vi "SaccadeAnalyser - Main.vi"(8 "error in (no error)":errorcluster, 11 "Data IN":T3={"Impulse Positions"=[{"Start"=5471, "End"=5813, "Impulse Plane"=enum."Yaw", "Impulse Direction +ve?"=FALSE, "Time offset"=0, "Amplitude offset"=0.0}, {"Start"=6974, "End"=7325, "Impulse Plane"=enum."Yaw", "Impulse Direction +ve?"=TRUE, "Time offset"=0, "Amplitude offset"=0.0}, {"Start"=7641, "End"=7980, "Impulse Plane"=enum."Yaw", "Impulse Direction +ve?"=FALSE, "Time offset"=0, "Amplitude offset"=0.0}, {"Start"=9060, "End"=9400, "Impulse Plane"=enum."Yaw", "Impulse Direction +ve?"=FALSE, "Time offset"=0, "Amplitude offset"=0.0}, {"Start"=9938, "End"=10282, "Impulse Plane"=enum."Yaw", "Impulse Direction +ve?"=FALSE, "Time offset"=0, "Amplitude offset"=0.0}, {"Start"=10800, "End"=11142, "Impulse Plane"=enum."Yaw", "Impulse Direction +ve?"=FALSE, "Time offset"=0, "Amplitude offset"=0.0}, {"Start"=11602, "End"=11942, "Impulse Plane"=enum."Yaw", "Impulse Direction +ve?"=TRUE, "Time offset"=0, "Amplitude offset"=0.0}, {"Start"=12449, "End"=12790, "Impulse Plane"=enum."Yaw", "Impulse Direction +ve?"=TRUE, "Time offset"=0, "Amplitude offset"=0.0}, {"Start"=13310, "End"=13653, "Impulse Plane"=enum."Yaw", "Impulse Direction +ve?"=TRUE, "Time offset"=0, "Amplitude offset"=0.0}, {"Start"=14191, "End"=14535, "Impulse Plane"=enum."Yaw", "Impulse Direction +ve?"=TRUE, "Time offset"=0, "Amplitude offset"=0.0}, {"Start"=15040, "End"=15380, "Impulse Plane"=enum."Yaw", "Impulse Direction +ve?"=FALSE, "Time offset"=0, "Amplitude offset"=0.0}, {"Start"=16780, "End"=17124, "Impulse Plane"=enum."Yaw", "Impulse Direction +ve?"=TRUE, "Time offset"=0, "Amplitude offset"=0.0}, {"Start"=17572, "End"=17913, "Impulse Plane"=enum."Yaw", "Impulse Direction +ve?"=FALSE, "Time offset"=0, "Amplitude offset"=0.0}, {"Start"=18369, "End"=18713, "Impulse Plane"=enum."Yaw", "Impulse Direction +ve?"=FALSE, "Time offset"=0, "Amplitude offset"=0.0}, {"Start"=19174, "End"=19519, "Impulse Plane"=enum."Yaw", "Impulse Direction +ve?"=FALSE, "Time offset"=0, "Amplitude offset"=0.0}, {"Start"=19928, "End"=20270, "Impulse Plane"=enum."Yaw", "Impulse Direction +ve?"=TRUE, "Time offset"=0, "Amplitude offset"=0.0}, {"Start"=20762, "End"=21121, "Impulse Plane"=enum."Yaw", "Impulse Direction +ve?"=FALSE, "Time offset"=0, "Amplitude offset"=0.0}, {"Start"=21554, "End"=21888, "Impulse Plane"=enum."Yaw", "Impulse Direction +ve?"=FALSE, "Time offset"=0, "Amplitude offset"=0.0}, {"Start"=22293, "End"=22639, "Impulse Plane"=enum."Yaw", "Impulse Direction +ve?"=TRUE, "Time offset"=0, "Amplitude offset"=0.0}, {"Start"=23109, "End"=23464, "Impulse Plane"=enum."Yaw", "Impulse Direction +ve?"=TRUE, "Time offset"=0, "Amplitude offset"=0.0}, {"Start"=23868, "End"=24215, "Impulse Plane"=enum."Yaw", "Impulse Direction +ve?"=TRUE, "Time offset"=0, "Amplitude offset"=0.0}, {"Start"=24643, "End"=24992, "Impulse Plane"=enum."Yaw", "Impulse Direction +ve?"=FALSE, "Time offset"=0, "Amplitude offset"=0.0}, {"Start"=25685, "End"=26023, "Impulse Plane"=enum."Yaw", "Impulse Direction +ve?"=FALSE, "Time offset"=0, "Amplitude offset"=0.0}, {"Start"=26431, "End"=26768, "Impulse Plane"=enum."Yaw", "Impulse Direction +ve?"=FALSE, "Time offset"=0, "Amplitude offset"=0.0}, {"Start"=27251, "End"=27595, "Impulse Plane"=enum."Yaw", "Impulse Direction +ve?"=FALSE, "Time offset"=0, "Amplitude offset"=0.0}, {"Start"=28832, "End"=29180, "Impulse Plane"=enum."Yaw", "Impulse Direction +ve?"=TRUE, "Time offset"=0, "Amplitude offset"=0.0}, {"Start"=31028, "End"=31383, "Impulse Plane"=enum."LARP", "Impulse Direction +ve?"=FALSE, "Time offset"=0, "Amplitude offset"=0.0}, {"Start"=32603, "End"=32936, "Impulse Plane"=enum."LARP", "Impulse Direction +ve?"=TRUE, "Time offset"=0, "Amplitude offset"=0.0}, {"Start"=33445, "End"=33779, "Impulse Plane"=enum."LARP", "Impulse Direction +ve?"=TRUE, "Time offset"=0, "Amplitude offset"=0.0}, {"Start"=34276, "End"=34629, "Impulse Plane"=enum."LARP", "Impulse Direction +ve?"=FALSE, "Time offset"=0, "Amplitude offset"=0.0}, {"Start"=35114, "End"=35460, "Impulse Plane"=enum."LARP", "Impulse Direction +ve?"=FALSE, "Time offset"=0, "Amplitude offset"=0.0}, {"Start"=35981, "End"=36324, "Impulse Plane"=enum."LARP", "Impulse Direction +ve?"=TRUE, "Time offset"=0, "Amplitude offset"=0.0}, {"Start"=36920, "End"=37249, "Impulse Plane"=enum."LARP", "Impulse Direction +ve?"=TRUE, "Time offset"=0, "Amplitude offset"=0.0}, {"Start"=37988, "End"=38322, "Impulse Plane"=enum."LARP", "Impulse Direction +ve?"=TRUE, "Time offset"=0, "Amplitude offset"=0.0}, {"Start"=38964, "End"=39324, "Impulse Plane"=enum."LARP", "Impulse Direction +ve?"=FALSE, "Time offset"=0, "Amplitude offset"=0.0}, {"Start"=39948, "End"=40284, "Impulse Plane"=enum."LARP", "Impulse Direction +ve?"=TRUE, "Time offset"=0, "Amplitude offset"=0.0}, {"Start"=40958, "End"=41293, "Impulse Plane"=enum."LARP", "Impulse Direction +ve?"=TRUE, "Time offset"=0, "Amplitude offset"=0.0}, {"Start"=41899, "End"=42229, "Impulse Plane"=enum."LARP", "Impulse Direction +ve?"=TRUE, "Time offset"=0, "Amplitude offset"=0.0}, {"Start"=42801, "End"=43154, "Impulse Plane"=enum."LARP", "Impulse Direction +ve?"=FALSE, "Time offset"=0, "Amplitude offset"=0.0}, {"Start"=43641, "End"=43980, "Impulse Plane"=enum."LARP", "Impulse Direction +ve?"=TRUE, "Time offset"=0, "Amplitude offset"=0.0}, {"Start"=44466, "End"=44821, "Impulse Plane"=enum."LARP", "Impulse Direction +ve?"=FALSE, "Time offset"=0, "Amplitude offset"=0.0}, {"Start"=45388, "End"=45722, "Impulse Plane"=enum."LARP", "Impulse Direction +ve?"=TRUE, "Time offset"=0, "Amplitude offset"=0.0}, {"Start"=46149, "End"=46510, "Impulse Plane"=enum."LARP", "Impulse Direction +ve?"=FALSE, "Time offset"=0, "Amplitude offset"=0.0}, {"Start"=47874, "End"=48206, "Impulse Plane"=enum."LARP", "Impulse Direction +ve?"=TRUE, "Time offset"=0, "Amplitude offset"=0.0}, {"Start"=50143, "End"=50479, "Impulse Plane"=enum."RALP", "Impulse Direction +ve?"=TRUE, "Time offset"=0, "Amplitude offset"=0.0}, {"Start"=50976, "End"=51310, "Impulse Plane"=enum."RALP", "Impulse Direction +ve?"=FALSE, "Time offset"=0, "Amplitude offset"=0.0}, {"Start"=51892, "End"=52226, "Impulse Plane"=enum."RALP", "Impulse Direction +ve?"=FALSE, "Time offset"=0, "Amplitude offset"=0.0}, {"Start"=52839, "End"=53171, "Impulse Plane"=enum."RALP", "Impulse Direction +ve?"=FALSE, "Time offset"=0, "Amplitude offset"=0.0}, {"Start"=53676, "End"=54012, "Impulse Plane"=enum."RALP", "Impulse Direction +ve?"=TRUE, "Time offset"=0, "Amplitude offset"=0.0}, {"Start"=54530, "End"=54877, "Impulse Plane"=enum."RALP", "Impulse Direction +ve?"=FALSE, "Time offset"=0, "Amplitude offset"=0.0}, {"Start"=55371, "End"=55711, "Impulse Plane"=enum."RALP", "Impulse Direction +ve?"=TRUE, "Time offset"=0, "Amplitude offset"=0.0}, {"Start"=56153, "End"=56482, "Impulse Plane"=enum."RALP", "Impulse Direction +ve?"=FALSE, "Time offset"=0, "Amplitude offset"=0.0}, {"Start"=57053, "End"=57390, "Impulse Plane"=enum."RALP", "Impulse Direction +ve?"=FALSE, "Time offset"=0, "Amplitude offset"=0.0}, {"Start"=57954, "End"=58292, "Impulse Plane"=enum."RALP", "Impulse Direction +ve?"=FALSE, "Time offset"=0, "Amplitude offset"=0.0}, {"Start"=58794, "End"=59130, "Impulse Plane"=enum."RALP", "Impulse Direction +ve?"=TRUE, "Time offset"=0, "Amplitude offset"=0.0}, {"Start"=59587, "End"=59931, "Impulse Plane"=enum."RALP", "Impulse Direction +ve?"=TRUE, "Time offset"=0, "Amplitude offset"=0.0}, {"Start"=60399, "End"=60744, "Impulse Plane"=enum."RALP", "Impulse Direction +ve?"=FALSE, "Time offset"=0, "Amplitude offset"=0.0}, {"Start"=61218, "End"=61559, "Impulse Plane"=enum."RALP", "Impulse Direction +ve?"=FALSE, "Time offset"=0, "Amplitude offset"=0.0}, {"Start"=62100, "End"=62442, "Impulse Plane"=enum."RALP", "Impulse Direction +ve?"=FALSE, "Time offset"=0, "Amplitude offset"=0.0}, {"Start"=62989, "End"=63322, "Impulse Plane"=enum."RALP", "Impulse Direction +ve?"=FALSE, "Time offset"=0, "Amplitude offset"=0.0}, {"Start"=63787, "End"=64136, "Impulse Plane"=enum."RALP", "Impulse Direction +ve?"=TRUE, "Time offset"=0, "Amplitude offset"=0.0}, {"Start"=64603, "End"=64953, "Impulse Plane"=enum."RALP", "Impulse Direction +ve?"=FALSE, "Time offset"=0, "Amplitude offset"=0.0}, {"Start"=65462, "End"=65795, "Impulse Plane"=enum."RALP", "Impulse Direction +ve?"=FALSE, "Time offset"=0, "Amplitude offset"=0.0}, {"Start"=66308, "End"=66645, "Impulse Plane"=enum."RALP", "Impulse Direction +ve?"=FALSE, "Time offset"=0, "Amplitude offset"=0.0}, {"Start"=67052, "End"=67402, "Impulse Plane"=enum."RALP", "Impulse Direction +ve?"=TRUE, "Time offset"=0, "Amplitude offset"=0.0}], "No. Imp"=15, "Parameter Time Series"=[{"time offset"=0.0, "Offset"=0.0, "Gain"=1.0, "inverse"=FALSE, "filter data"=FALSE, "dots"=FALSE, "interpolate"=FALSE, "List 1"=5, "Color Box"=6618880, "Boolean"=TRUE}, {"time offset"=0.0, "Offset"=0.0, "Gain"=1.0, "inverse"=FALSE, "filter data"=FALSE, "dots"=FALSE, "interpolate"=FALSE, "List 1"=6, "Color Box"=6618880, "Boolean"=FALSE}, {"time offset"=0.0, "Offset"=0.0, "Gain"=1.0, "inverse"=FALSE, "filter data"=FALSE, "dots"=FALSE, "interpolate"=FALSE, "List 1"=7, "Color Box"=6618880, "Boolean"=FALSE}, {"time offset"=0.0, "Offset"=0.0, "Gain"=1.0, "inverse"=FALSE, "filter data"=FALSE, "dots"=FALSE, "interpolate"=FALSE, "List 1"=13, "Color Box"=16777224, "Boolean"=TRUE}, {"time offset"=0.0, "Offset"=0.0, "Gain"=1.0, "inverse"=FALSE, "filter data"=FALSE, "dots"=FALSE, "interpolate"=FALSE, "List 1"=14, "Color Box"=16777224, "Boolean"=FALSE}, {"time offset"=0.0, "Offset"=0.0, "Gain"=1.0, "inverse"=FALSE, "filter data"=FALSE, "dots"=FALSE, "interpolate"=FALSE, "List 1"=15, "Color Box"=16777224, "Boolean"=FALSE}], "Parameter Impuls Series"=[{"Color"=6618880, "Visible"=TRUE, "Channel"=1, "Invert"=FALSE, "Desaccade"=FALSE, "Offset"=0.0, "Gain"=1.0}, {"Color"=6618880, "Visible"=FALSE, "Channel"=6, "Invert"=FALSE, "Desaccade"=FALSE, "Offset"=0.0, "Gain"=1.0}, {"Color"=6618880, "Visible"=FALSE, "Channel"=7, "Invert"=FALSE, "Desaccade"=FALSE, "Offset"=0.0, "Gain"=1.0}, {"Color"=16777224, "Visible"=TRUE, "Channel"=13, "Invert"=FALSE, "Desaccade"=FALSE, "Offset"=0.0, "Gain"=1.0}, {"Color"=16777224, "Visible"=FALSE, "Channel"=14, "Invert"=FALSE, "Desaccade"=FALSE, "Offset"=0.0, "Gain"=1.0}, {"Color"=16777224, "Visible"=FALSE, "Channel"=15, "Invert"=FALSE, "Desaccade"=FALSE, "Offset"=0.0, "Gain"=1.0}], "Experiment Parameters"={"Freq"=0.0, "Vel"=0, "Acc"=0, "Stimulus"="Head Impulse"}, "Autosort File"=refnum, "Data File"={"Data Channels"=array34x71049[2415666 elements], "Sample Rate"=500, "Channel List"=["Hz Position-in-Head", "Hz Velocity-in-Head", "Hy Position-in-Head", "Hy Velocity-in-Head", "Hx Position-in-Head", "Hx Velocity-in-Head", "Hl Velocity-in-Head", "Hr Velocity-in-Head", "Lx Position-in-Head", "Ly Position-in-Head", "Lz Position-in-Head", "Lx Velocity-in-Head", "Ly Velocity-in-Head", "Lz Velocity-in-Head", "Ll Velocity-in-Head", "Lr Velocity-in-Head", "Rx Position-in-Head", "Ry Position-in-Head", "Rz Position-in-Head", "Rx Velocity-in-Head", "Ry Velocity-in-Head", "Rz Velocity-in-Head", "Rl Velocity-in-Head", "Rr Velocity-in-Head", "Target on/off", "aux input 1", "aux input 2", " ", "", "", "", "Target Hor", "Target Ver", ""]}, "Experiment data path"=path "C:/Users/w.figtree/Desktop/Coils Data/3", "Image data path"=path "/Macintosh HD/Users/patrick/Studium/Diploma Thesis/Data Analysis", "LVS data path"=path "/Macintosh HD/Users/patrick/Studium/Diploma Thesis/Data Analysis", "Raw copy path"=path "/Macintosh HD/Users/patrick/Studium/Diploma Thesis/Data Analysis", "filename"="passive_lvs.lvs", "desaccading parameters"={"Tolerance"=3, "Acc Range"=7000.0, "Sample Rate"=500, "Impulse Plane 2"=enum."Yaw", "Impulse dir"=FALSE}, "Experiment Parameters 2"={"Subject"="SE Trial Short Term", "Strain"="", "Rotation plane"="", "Experimenter"=" ", "Trial"=0.0, "Time"=0.0}, "Excel"={"Excel._Application"=refnum, "Use Excel"=TRUE, "Worksheet SINE"=refnum, "Row SINE"=0, "Worksheet TRANS"=refnum, "Row TRANS"=0}, "Session Config File"=refnum, "Autosort Parameter Set"=4, "EMA Version"="EMA 2016a", "desacc "={"Threshold 1 [Acc]"=7000.0, "Threshold 2 [% of TH1]"=60, "tolerance"=3, "Search WD "=0.1, " always use TH2"=FALSE, "Range"=3.0, "Max time"=120.0, "Min time"=20.0, "Velocity Threshold"=150}, "Cycle Nr for Saccades"={"POS"=0, "NEG"=0}, "calibration name"="u_calibration_1_p00001s001_calib.mat", "Excel"=refnum} {"Parameter Time Series"."time offset" format="%.3f"; "Parameter Time Series"."Gain" format="%.1f"; "Parameter Time Series"."Offset" format="%.1f"; "Parameter Time Series"."List 1" items=["Motor-Pos", "Motor-Vel", "Lx Position-in-Head", "Ly Position-in-Head", "Lz Position-in-Head", "Lx Velocity-in-Head", "Ly Velocity-in-Head", "Lz Velocity-in-Head", "Ll Velocity-in-Head", "Lr Velocity-in-Head", "Lx Accel-in-Head", "Ly Accel-in-Head", "Lz Accel-in-Head", "Rx Position-in-Head", "Ry Position-in-Head", "Rz Position-in-Head", "Rx Velocity-in-Head", "Ry Velocity-in-Head", "Rz Velocity-in-Head", "Rl Velocity-in-Head", "Rr Velocity-in-Head", "Rx Accel-in-Head", "Ry Accel-in-Head", "Rz Accel-in-Head", "Global Trigger", "", "", ""]; "Parameter Impuls Series"."Gain" format="%.1f"; "Parameter Impuls Series"."Offset" format="%.1f"}) -> (0 "error out":errorcluster, 3 "Data OUT":T3={"Impulse Positions"=[{"Start"=5471, "End"=5813, "Impulse Plane"=enum."Yaw", "Impulse Direction +ve?"=FALSE, "Time offset"=0, "Amplitude offset"=0.0}, {"Start"=6974, "End"=7325, "Impulse Plane"=enum."Yaw", "Impulse Direction +ve?"=TRUE, "Time offset"=0, "Amplitude offset"=0.0}, {"Start"=7641, "End"=7980, "Impulse Plane"=enum."Yaw", "Impulse Direction +ve?"=FALSE, "Time offset"=0, "Amplitude offset"=0.0}, {"Start"=9060, "End"=9400, "Impulse Plane"=enum."Yaw", "Impulse Direction +ve?"=FALSE, "Time offset"=0, "Amplitude offset"=0.0}, {"Start"=9938, "End"=10282, "Impulse Plane"=enum."Yaw", "Impulse Direction +ve?"=FALSE, "Time offset"=0, "Amplitude offset"=0.0}, {"Start"=10800, "End"=11142, "Impulse Plane"=enum."Yaw", "Impulse Direction +ve?"=FALSE, "Time offset"=0, "Amplitude offset"=0.0}, {"Start"=11602, "End"=11942, "Impulse Plane"=enum."Yaw", "Impulse Direction +ve?"=TRUE, "Time offset"=0, "Amplitude offset"=0.0}, {"Start"=12449, "End"=12790, "Impulse Plane"=enum."Yaw", "Impulse Direction +ve?"=TRUE, "Time offset"=0, "Amplitude offset"=0.0}, {"Start"=13310, "End"=13653, "Impulse Plane"=enum."Yaw", "Impulse Direction +ve?"=TRUE, "Time offset"=0, "Amplitude offset"=0.0}, {"Start"=14191, "End"=14535, "Impulse Plane"=enum."Yaw", "Impulse Direction +ve?"=TRUE, "Time offset"=0, "Amplitude offset"=0.0}, {"Start"=15040, "End"=15380, "Impulse Plane"=enum."Yaw", "Impulse Direction +ve?"=FALSE, "Time offset"=0, "Amplitude offset"=0.0}, {"Start"=16780, "End"=17124, "Impulse Plane"=enum."Yaw", "Impulse Direction +ve?"=TRUE, "Time offset"=0, "Amplitude offset"=0.0}, {"Start"=17572, "End"=17913, "Impulse Plane"=enum."Yaw", "Impulse Direction +ve?"=FALSE, "Time offset"=0, "Amplitude offset"=0.0}, {"Start"=18369, "End"=18713, "Impulse Plane"=enum."Yaw", "Impulse Direction +ve?"=FALSE, "Time offset"=0, "Amplitude offset"=0.0}, {"Start"=19174, "End"=19519, "Impulse Plane"=enum."Yaw", "Impulse Direction +ve?"=FALSE, "Time offset"=0, "Amplitude offset"=0.0}, {"Start"=19928, "End"=20270, "Impulse Plane"=enum."Yaw", "Impulse Direction +ve?"=TRUE, "Time offset"=0, "Amplitude offset"=0.0}, {"Start"=20762, "End"=21121, "Impulse Plane"=enum."Yaw", "Impulse Direction +ve?"=FALSE, "Time offset"=0, "Amplitude offset"=0.0}, {"Start"=21554, "End"=21888, "Impulse Plane"=enum."Yaw", "Impulse Direction +ve?"=FALSE, "Time offset"=0, "Amplitude offset"=0.0}, {"Start"=22293, "End"=22639, "Impulse Plane"=enum."Yaw", "Impulse Direction +ve?"=TRUE, "Time offset"=0, "Amplitude offset"=0.0}, {"Start"=23109, "End"=23464, "Impulse Plane"=enum."Yaw", "Impulse Direction +ve?"=TRUE, "Time offset"=0, "Amplitude offset"=0.0}, {"Start"=23868, "End"=24215, "Impulse Plane"=enum."Yaw", "Impulse Direction +ve?"=TRUE, "Time offset"=0, "Amplitude offset"=0.0}, {"Start"=24643, "End"=24992, "Impulse Plane"=enum."Yaw", "Impulse Direction +ve?"=FALSE, "Time offset"=0, "Amplitude offset"=0.0}, {"Start"=25685, "End"=26023, "Impulse Plane"=enum."Yaw", "Impulse Direction +ve?"=FALSE, "Time offset"=0, "Amplitude offset"=0.0}, {"Start"=26431, "End"=26768, "Impulse Plane"=enum."Yaw", "Impulse Direction +ve?"=FALSE, "Time offset"=0, "Amplitude offset"=0.0}, {"Start"=27251, "End"=27595, "Impulse Plane"=enum."Yaw", "Impulse Direction +ve?"=FALSE, "Time offset"=0, "Amplitude offset"=0.0}, {"Start"=28832, "End"=29180, "Impulse Plane"=enum."Yaw", "Impulse Direction +ve?"=TRUE, "Time offset"=0, "Amplitude offset"=0.0}, {"Start"=31028, "End"=31383, "Impulse Plane"=enum."LARP", "Impulse Direction +ve?"=FALSE, "Time offset"=0, "Amplitude offset"=0.0}, {"Start"=32603, "End"=32936, "Impulse Plane"=enum."LARP", "Impulse Direction +ve?"=TRUE, "Time offset"=0, "Amplitude offset"=0.0}, {"Start"=33445, "End"=33779, "Impulse Plane"=enum."LARP", "Impulse Direction +ve?"=TRUE, "Time offset"=0, "Amplitude offset"=0.0}, {"Start"=34276, "End"=34629, "Impulse Plane"=enum."LARP", "Impulse Direction +ve?"=FALSE, "Time offset"=0, "Amplitude offset"=0.0}, {"Start"=35114, "End"=35460, "Impulse Plane"=enum."LARP", "Impulse Direction +ve?"=FALSE, "Time offset"=0, "Amplitude offset"=0.0}, {"Start"=35981, "End"=36324, "Impulse Plane"=enum."LARP", "Impulse Direction +ve?"=TRUE, "Time offset"=0, "Amplitude offset"=0.0}, {"Start"=36920, "End"=37249, "Impulse Plane"=enum."LARP", "Impulse Direction +ve?"=TRUE, "Time offset"=0, "Amplitude offset"=0.0}, {"Start"=37988, "End"=38322, "Impulse Plane"=enum."LARP", "Impulse Direction +ve?"=TRUE, "Time offset"=0, "Amplitude offset"=0.0}, {"Start"=38964, "End"=39324, "Impulse Plane"=enum."LARP", "Impulse Direction +ve?"=FALSE, "Time offset"=0, "Amplitude offset"=0.0}, {"Start"=39948, "End"=40284, "Impulse Plane"=enum."LARP", "Impulse Direction +ve?"=TRUE, "Time offset"=0, "Amplitude offset"=0.0}, {"Start"=40958, "End"=41293, "Impulse Plane"=enum."LARP", "Impulse Direction +ve?"=TRUE, "Time offset"=0, "Amplitude offset"=0.0}, {"Start"=41899, "End"=42229, "Impulse Plane"=enum."LARP", "Impulse Direction +ve?"=TRUE, "Time offset"=0, "Amplitude offset"=0.0}, {"Start"=42801, "End"=43154, "Impulse Plane"=enum."LARP", "Impulse Direction +ve?"=FALSE, "Time offset"=0, "Amplitude offset"=0.0}, {"Start"=43641, "End"=43980, "Impulse Plane"=enum."LARP", "Impulse Direction +ve?"=TRUE, "Time offset"=0, "Amplitude offset"=0.0}, {"Start"=44466, "End"=44821, "Impulse Plane"=enum."LARP", "Impulse Direction +ve?"=FALSE, "Time offset"=0, "Amplitude offset"=0.0}, {"Start"=45388, "End"=45722, "Impulse Plane"=enum."LARP", "Impulse Direction +ve?"=TRUE, "Time offset"=0, "Amplitude offset"=0.0}, {"Start"=46149, "End"=46510, "Impulse Plane"=enum."LARP", "Impulse Direction +ve?"=FALSE, "Time offset"=0, "Amplitude offset"=0.0}, {"Start"=47874, "End"=48206, "Impulse Plane"=enum."LARP", "Impulse Direction +ve?"=TRUE, "Time offset"=0, "Amplitude offset"=0.0}, {"Start"=50143, "End"=50479, "Impulse Plane"=enum."RALP", "Impulse Direction +ve?"=TRUE, "Time offset"=0, "Amplitude offset"=0.0}, {"Start"=50976, "End"=51310, "Impulse Plane"=enum."RALP", "Impulse Direction +ve?"=FALSE, "Time offset"=0, "Amplitude offset"=0.0}, {"Start"=51892, "End"=52226, "Impulse Plane"=enum."RALP", "Impulse Direction +ve?"=FALSE, "Time offset"=0, "Amplitude offset"=0.0}, {"Start"=52839, "End"=53171, "Impulse Plane"=enum."RALP", "Impulse Direction +ve?"=FALSE, "Time offset"=0, "Amplitude offset"=0.0}, {"Start"=53676, "End"=54012, "Impulse Plane"=enum."RALP", "Impulse Direction +ve?"=TRUE, "Time offset"=0, "Amplitude offset"=0.0}, {"Start"=54530, "End"=54877, "Impulse Plane"=enum."RALP", "Impulse Direction +ve?"=FALSE, "Time offset"=0, "Amplitude offset"=0.0}, {"Start"=55371, "End"=55711, "Impulse Plane"=enum."RALP", "Impulse Direction +ve?"=TRUE, "Time offset"=0, "Amplitude offset"=0.0}, {"Start" (continued)
-2.8883541530445154, -3.516148902040583, -3.9328497535351947, -4.074952205861335, -3.9264797477619506, -3.5235880515318287, -2.9445085168642864, -2.2825465992610874, -1.6346125625456331, -1.0868528306011866, -0.6892793448005747, -0.4514233697419858, -0.34772068565764536, -0.33144239906252126, -0.35236114149875597, -0.368063510951562, -0.3536819185740605, -0.30593479455420614, -0.24082377197891836, -0.18644123364218523, -0.17235627530367026, -0.21733087397872697, -0.32105772809018474, -0.46282725799962887, -0.6013468636250685, -0.681029316469846, -0.6453789933024492, -0.4464563108376538, -0.05711793420641298, 0.5195291111813729, 1.24460428742947, 2.0409035585143225, 2.8071974605790397, 3.4374680689449324, 3.8362889910863416, 3.936137192044335, 3.7133156246449173, 3.1962055823983055, 2.4645339267973876, 1.6323339053855144, 0.8281887193758093, 0.17895741983626667, -0.21794588340546106, -0.3149797233911795, -0.1208780028004468, 0.3010279142001131, 0.8466949029935436, 1.3889212429561213, 1.8001793228350753, 1.9794383864747012, 1.872001773439452, 1.4802280655606248, 0.8678649317771643, 0.15408792967003448, -0.5121669703474789, -0.9809448053789069, -1.1274894734750562, -0.884225278628704, -0.2573077848332693, 0.6755098232318858, 1.769203172647637, 2.838433340284629, 3.7048996921835853, 4.232291904461003, 4.349215560850677, 4.067996077468677, 3.4852532459476757, 2.7551766825107906, 2.0545001121225317, 1.5433035301714788, 1.3340545644670074, 1.4757615276377378, 1.943838013156551, 2.6492549395734972, 3.464119840160972, 4.249700389985186, 4.879134744661279, 5.264037307615373, 5.370444593979055, 5.218155701632909, 4.875603814292236, 4.438467035967314, 4.0082473127717995, 3.6799618353064303, 3.5304971825025597, 3.59372264810927, 3.8502768373813416, 4.247704826083448, 4.709723464311016]}, {[0.0, 2.0, 4.0, 6.0, 8.0, 10.0, 12.0, 14.0, 16.0, 18.000000000000004, 20.0, 22.0, 24.0, 26.000000000000004, 28.0, 30.0, 32.0, 34.0, 36.00000000000001, 38.0, 40.0, 42.0, 44.0, 46.0, 48.0, 50.0, 52.00000000000001, 54.0, 56.0, 58.0, 60.0, 62.0, 64.0, 66.0, 68.0, 70.0, 72.00000000000001, 74.0, 76.0, 78.0, 80.0, 82.0, 84.0, 86.0, 88.0, 90.0, 92.0, 94.0, 96.0, 98.0, 100.0, 102.00000000000001, 104.00000000000001, 106.0, 108.0, 110.0, 112.0, 114.0, 116.0, 118.00000000000001, 120.0, 122.0, 124.0, 126.0, 128.0, 130.0, 132.0, 134.0, 136.0, 138.0, 140.0, 142.00000000000003, 144.00000000000003, 146.0, 148.0, 150.0, 152.0, 154.0, 156.0, 158.0, 160.0, 162.0, 164.0, 166.0, 168.0, 170.0, 172.0, 174.00000000000003, 176.0, 178.0, 180.0, 182.0, 184.0, 186.0, 188.0, 190.0, 192.0, 194.0, 196.0, 198.0, 200.0, 202.0, 204.00000000000003, 206.00000000000003, 208.00000000000003, 210.0, 212.0, 214.0, 216.0, 218.0, 220.0, 222.0, 224.0, 226.0, 228.0, 230.0, 232.0, 234.0, 236.00000000000003, 238.00000000000003, 240.0, 242.0, 244.0, 246.0, 248.0, 250.0, 252.0, 254.0, 256.0, 258.0, 260.0, 262.0, 264.0, 266.0, 268.0, 270.0, 272.0, 274.0, 276.0, 278.0, 280.0, 282.0, 284.00000000000006, 286.00000000000006, 288.00000000000006, 290.0, 292.0, 294.0, 296.0, 298.0, 300.0, 302.0, 304.0, 306.0, 308.0, 310.0, 312.0, 314.0, 316.0, 318.0, 320.0, 322.0, 324.0, 326.0, 328.0, 330.0, 332.0, 334.0, 336.0, 338.0, 340.0, 342.0, 344.0, 346.00000000000006, 348.00000000000006, 350.00000000000006, 352.0, 354.0, 356.0, 358.0, 360.0, 362.0, 364.0, 366.0, 368.0, 370.0, 372.0, 374.0, 376.0, 378.0, 380.0, 382.0, 384.0, 386.0, 388.0, 390.0, 392.0, 394.0, 396.0, 398.0, 400.0, 402.0, 404.0, 406.0, 408.00000000000006, 410.00000000000006, 412.00000000000006, 414.00000000000006, 416.00000000000006, 418.0, 420.0, 422.0, 424.0, 426.0, 428.0, 430.0, 432.0, 434.0, 436.0, 438.0, 440.0, 442.0, 444.0, 446.0, 448.0, 450.0, 452.0, 454.0, 456.0, 458.0, 460.0, 462.0, 464.0, 466.0, 468.0, 470.00000000000006, 472.00000000000006, 474.00000000000006, 476.00000000000006, 478.00000000000006, 480.0, 482.0, 484.0, 486.0, 488.0, 490.0, 492.0, 494.0, 496.0, 498.0, 500.0, 502.0, 504.0, 506.0, 508.0, 510.0, 512.0, 514.0, 516.0, 518.0, 520.0, 522.0, 524.0, 526.0, 528.0, 530.0, 532.0, 534.0, 536.0, 538.0, 540.0, 542.0, 544.0, 546.0, 548.0, 550.0, 552.0, 554.0, 556.0, 558.0, 560.0, 562.0, 564.0, 566.0000000000001, 568.0000000000001, 570.0000000000001, 572.0000000000001, 574.0000000000001, 576.0000000000001, 578.0, 580.0, 582.0, 584.0, 586.0, 588.0, 590.0, 592.0, 594.0, 596.0, 598.0, 600.0, 602.0, 604.0, 606.0, 608.0, 610.0, 612.0, 614.0, 616.0, 618.0, 620.0, 622.0, 624.0, 626.0, 628.0, 630.0, 632.0, 634.0, 636.0, 638.0, 640.0, 642.0, 644.0, 646.0, 648.0, 650.0, 652.0, 654.0, 656.0, 658.0, 660.0, 662.0, 664.0, 666.0, 668.0], [-0.9334894772952316, 0.1801268761223227, 1.6003470306951726, 3.153831134806954, 4.462794878724324, 4.97211069807356, 4.036974033253972, 1.061742180594367, -4.321167540703003, -12.102974473794017, -21.819347732352327, -32.540042582787876, -42.96163513491041, -51.61678053063674, -57.122252746441816, -58.43889613683768, -55.095052084056775, -47.28747209206602, -35.87076591841188, -22.22033959221386, -7.997162936365397, 5.123758485672756, 15.726987142783598, 22.86581407251021, 26.16840202466106, 25.83579153913346, 22.54156839413768, 17.26164162751238, 11.073942357029717, 4.9794288053074, -0.23849491571313752, -4.098790026284233, -6.4259588883232635, -7.308484018772553, -7.025538729742294, -5.9569308755366475, -4.499287428317563, -2.996388304103705, -1.702781426779054, -0.7660627372425493, -0.23182136516608742, -0.06494318297779444, -0.1675368789302516, -0.40660179816048625, -0.6442032640935491, -0.75885792027574, -0.6637955445910451, -0.3198247987273777, 0.25481799202614486, 0.9828310807590925, 1.7418709355694801, 2.3838213472274434, 2.7723253745745815, 2.81627930193372, 2.4838470040047644, 1.8289475281337975, 0.9788023972195348, 0.09480395200899672, -0.6487174954960242, -1.1044616210506086, -1.2009175258855735, -0.9550491005804087, -0.4476054105625138, 0.19430988816920614, 0.8342358428617173, 1.3820041868156303, 1.811438380233771, 2.1600586820990606, 2.5203383690122863, 3.007130016971932, 3.714133573254492, 4.684538146497915, 5.904472546107545, 7.31141890036135, 8.817433946059205, 10.340183047257561, 11.833990195220093, 13.307826887863264, 14.82279250346561, 16.48338589999716, 18.398448358908524, 20.64720578019333, 23.275776374704144, 26.282069902940513, 29.623866571210993, 33.23121815954027, 37.022577537184134, 40.933861626605854, 44.92341083367323, 48.977769503983254, 53.10255808997472, 57.31293200910059, 61.641364731262634, 66.12197602278071, 70.77588871120423, 75.61308429636848, 80.62653268616691, 85.78676107670987, 91.03553459263824, 96.29409592735007, 101.48333369820773, 106.52886617072996, 111.37740389502292, 116.01947167443313, 120.48739524556416, 124.84001094233074, 129.1521691932076, 133.4901602423704, 137.88012392460402, 142.30017164297595, 146.6868525851271, 150.94371694046887, 154.96493425184485, 158.66918705594242, 162.0136112128972, 165.00302368924463, 167.6889936618766, 170.1399732648479, 172.42388911283476, 174.59194864876082, 176.65068233647204, 178.56059762526655, 180.25044857037415, 181.63380562077862, 182.6259785855574, 183.15471452874053, 183.17399509118056, 182.65865459204537, 181.59313761999684, 179.97073408550776, 177.77522338872325, 174.98724912180214, 171.5955451691914, 167.59569372935653, 163.0136611998637, 157.90995884182604, 152.36800745229903, 146.4885501798765, 140.38114201894598, 134.14835627984627, 127.86429952676306, 121.57142537085608, 115.29301533963887, 109.03754459247074, 102.81096990925926, 96.63539378751156, 90.5427036061671, 84.56850699787714, 78.7468659593296, 73.08832506520068, 67.57567167066148, 62.15665315872718, 56.73648067790759, 51.213306336744715, 45.5053657518873, 39.55793518034204, 33.37467323039037, 27.033914938813158, 20.671923830437372, 14.464194619968211, 8.6030681983396, 3.26183636017426, -1.443375473945356, -5.461423649645508, -8.806137363082733, -11.547667911787219, -13.788980955917005, -15.65126548395963, -17.239999767745942, -18.628355475006167, -19.862255020323055, -20.95332940558723, -21.89368326704327, -22.675220607148425, -23.297380238236382, -23.767966018157527, -24.098928341873194, -24.31117125728565, -24.427128043175212, -24.45575909528184, -24.393314175848772, -24.223828923103603, -23.926237104554602, -23.48791867551934, -22.90549868470649, -22.193920531019455, -21.39129147319717, -20.543427852789435, -19.694214229777813, -18.877041123326624, -18.102773683811797, -17.353664883725877, -16.58974194021117, -15.76268505154159, -14.822681580885476, -13.731469159982414, -12.480650096798229, -11.097015153148108, -9.63471978449036, -8.172406368248037, -6.800537407725622, -5.602907366224802, -4.645618806504073, -3.959792840430265, -3.540595838440085, -3.3467811584963973, -3.302221129527577, -3.3126019104870728, -3.2805911155766707, -3.12851529901644, -2.81907953972555, -2.3631322564936577, -1.8227593656953187, -1.299646490130245, -0.9176962720213462, -0.8021816964917609, -1.0490559905228913, -1.6966074457005087, -2.7071960196468963, -3.9796708607327593, -5.363887154712282, -6.674806686075243, -7.729898062533455, -8.388005815865553, -8.578502674610748, -8.306656293797122, -7.6500076555824865, -6.7510806469438, -5.785630277133685, -4.930387667691571, -4.340731190160524, -4.122500323387578, -4.31067226273608, -4.869055227280224, -5.697226571848775, -6.656858262673733, -7.6027724886940735, -8.397122141556054, -8.935264499281871, -9.167892297392665, -9.106974048521735, -8.815107448791384, -8.385949446059211, -7.921195009004617, -7.506045107570235, -7.19506753073141, -6.996064068390508, -6.8730002641486445, -6.766031511347408, -6.60819552351697, -6.352074966023138, -5.987730014405243, -5.538008698234154, -5.053804358977626, -4.6070463097324925, -4.267804730344441, -4.081663983188778, -4.062723321604938, -4.189394584998989, -4.406702517932528, -4.651794525673151, -4.870615088974423, -5.023561094636401, -5.08919179890909, -5.0620169068343674, -4.950395506820692, -4.759844626890361, -4.47978396480668, -4.087870297150788, -3.5695605496339615, -2.937629326655836, -2.2471495382904587, -1.6135331812473233, -1.206848808632663, -1.2153494406916945, -1.7865063418060716, -2.946522962811934, -4.522231629389672, -6.099356541635326, -7.033837566184765, -6.530522920748879, -3.7817473387038465, 1.850754719532537, 10.642426983685915, 22.365587411552568, 36.23501199222388, 50.94709617216887, 64.84101602206391, 76.17471628829185, 83.41922636843152, 85.51991298092757, 82.09980450239388, 73.53608919952723, 60.89872991717725, 45.758420318077484, 29.907265361805152, 15.058407133564199, 2.5737382904767507, -6.715899336652479, -12.57598159697483, -15.3246447501556, -15.686631915632411, -14.574916517929267, -12.872113276125042, -11.256596904519734, -10.087800141504514, -9.38898168546973, -8.931418503800682, -8.378381558333455, -7.455938221472304, -6.1149563875848845, -4.630479374884101, -3.6087389566511083, -3.8979759878801428, -6.418841896556859, -11.934085038616296, -20.81166991401699, -32.85800497539039, -47.25661341526123, -62.63483051980433, -77.2486679973641, -89.2682568442995, -97.1183555061835, -99.76622149223874, -96.90020663268331, -88.9882565902794, -77.18428314815168, -63.08714163333932, -48.44329847046076, -34.84976354959394, -23.500142815636288, -15.03908288349576, -9.553995446693445, -6.678386379629533]}, {[0.0, 2.0, 4.0, 6.0, 8.0, 10.0, 12.0, 14.0, 16.0, 18.000000000000004, 20.0, 22.0, 24.0, 26.000000000000004, 28.0, 30.0, 32.0, 34.0, 36.00000000000001, 38.0, 40.0, 42.0, 44.0, 46.0, 48.0, 50.0, 52.00000000000001, 54.0, 56.0, 58.0, 60.0, 62.0, 64.0, 66.0, 68.0, 70.0, 72.00000000000001, 74.0, 76.0, 78.0, 80.0, 82.0, 84.0, 86.0, 88.0, 90.0, 92.0, 94.0, 96.0, 98.0, 100.0, 102.00000000000001, 104.00000000000001, 106.0, 108.0, 110.0, 112.0, 114.0, 116.0, 118.00000000000001, 120.0, 122.0, 124.0, 126.0, 128.0, 130.0, 132.0, 134.0, 136.0, 138.0, 140.0, 142.00000000000003, 144.00000000000003, 146.0, 148.0, 150.0, 152.0, 154.0, 156.0, 158.0, 160.0, 162.0, 164.0, 166.0, 168.0, 170.0, 172.0, 174.00000000000003, 176.0, 178.0, 180.0, 182.0, 184.0, 186.0, 188.0, 190.0, 192.0, 194.0, 196.0, 198.0, 200.0, 202.0, 204.00000000000003, 206.00000000000003, 208.00000000000003, 210.0, 212.0, 214.0, 216.0, 218.0, 220.0, 222.0, 224.0, 226.0, 228.0, 230.0, 232.0, 234.0, 236.00000000000003, 238.00000000000003, 240.0, 242.0, 244.0, 246.0, 248.0, 250.0, 252.0, 254.0, 256.0, 258.0, 260.0, 262.0, 264.0, 266.0, 268.0, 270.0, 272.0, 274.0, 276.0, 278.0, 280.0, 282.0, 284.00000000000006, 286.00000000000006, 288.00000000000006, 290.0, 292.0, 294.0, 296.0, 298.0, 300.0, 302.0, 304.0, 306.0, 308.0, 310.0, 312.0, 314.0, 316.0, 318.0, 320.0, 322.0, 324.0, 326.0, 328.0, 330.0, 332.0, 334.0, 336.0, 338.0, 340.0, 342.0, 344.0, 346.00000000000006, 348.00000000000006, 350.00000000000006, 352.0, 354.0, 356.0, 358.0, 360.0, 362.0, 364.0, 366.0, 368.0, 370.0, 372.0, 374.0, 376.0, 378.0, 380.0, 382.0, 384.0, 386.0, 388.0, 390.0, 392.0, 394.0, 396.0, 398.0, 400.0, 402.0, 404.0, 406.0, 408.00000000000006, 410.00000000000006, 412.00000000000006, 414.00000000000006, 416.00000000000006, 418.0, 420.0, 422.0, 424.0, 426.0, 428.0, 430.0, 432.0, 434.0, 436.0, 438.0, 440.0, 442.0, 444.0, 446.0, 448.0, 450.0, 452.0, 454.0, 456.0, 458.0, 460.0, 462.0, 464.0, 466.0, 468.0, 470.00000000000006, 472.00000000000006, 474.00000000000006, 476.00000000000006, 478.00000000000006, 480.0, 482.0, 484.0, 486.0, 488.0, 490.0, 492.0, 494.0, 496.0, 498.0, 500.0, 502.0, 504.0, 506.0, 508.0, 510.0, 512.0, 514.0, 516.0, 518.0, 520.0, 522.0, 524.0, 526.0, 528.0, 530.0, 532.0, 534.0, 536.0, 538.0, 540.0, 542.0, 544.0, 546.0, 548.0, 550.0, 552.0, 554.0, 556.0, 558.0, 560.0, 562.0, 564.0, 566.0000000000001, 568.0000000000001, 570.0000000000001, 572.0000000000001, 574.0000000000001, 576.0000000000001, 578.0, 580.0, 582.0, 584.0, 586.0, 588.0, 590.0, 592.0, 594.0, 596.0, 598.0, 600.0, 602.0, 604.0, 606.0, 608.0, 610.0, 612.0, 614.0, 616.0, 618.0, 620.0, 622.0, 624.0, 626.0, 628.0, 630.0, 632.0, 634.0, 636.0, 638.0, 640.0, 642.0, 644.0, 646.0, 648.0, 650.0, 652.0, 654.0, 656.0, 658.0, 660.0, 662.0, 664.0, 666.0, 668.0], [-0.3359044865150098, -0.2260920816078409, -0.09756470825443042, 0.008658949479325884, 0.06732910891758981, 0.06807062686455723, 0.01821544705331335, -0.059601811260349136, -0.14347411386778575, -0.21765857664065513, -0.26957083645469027, -0.2898071738550543, -0.27729708714535395, -0.23676487915418964, -0.18093104483067135, -0.12538975405713382, -0.07680373613825453, -0.04321965675080519, -0.03058294007206741, -0.03823931058922003, -0.062066652926533905, -0.09131713108715145, -0.10928333240745913, -0.09573259382452481, -0.031040651821538923, 0.09991211191956784, 0.3027604182255834, 0.569849180154238, 0.8827491045923315, 1.2094834496529898, 1.5096805949425085, 1.7490166684012822, 1.8979592284586553, 1.937643616873436, 1.8684803481161545, 1.7070976500990742, 1.4834138145812015, 1.2366831266673348, 1.0079409691809322, 0.8312251781804393, 0.7297017909026405, 0.7082926692514193, 0.7463215838812411, 0.8035836326690542, 0.8279793883349749, 0.7655725418305352, 0.5708493147226708, 0.21520599350414082, -0.2944842529814382, -0.9130950028513514, -1.567593400869794, -2.163920747070543, -2.6112146044651636, -2.8428180918431383, -2.8255217303845104, -2.5773191979501524, -2.162601637296418, -1.6727164581037948, -1.213095823656574, -0.8837852845109531, -0.7554155059442453, -0.849680570099641, -1.1463103161130603, -1.594969229000521, -2.1304366583433483, -2.698804190840396, -3.265952257398339, -3.8226717629035223, -4.3903509507397445, -5.009842320487963, -5.72038578226646, -6.547185232526366, -7.500090811921922, -8.575161763669628, -9.762075389822414, -11.053767811142349, -12.460364891175711, -14.01320079725716, -15.754191611336893, -17.73739198870132, -20.00807515860909, -22.579611028115956, -25.44137263434334, -28.558668377305896, -31.87671494481618, -35.33355341287755, -38.87611458484757, -42.46966861641875, -46.10144373994499, -49.78491202475567, -53.544814213240194, -57.41234403003223, -61.43013207030185, -65.63105454094075, -70.02843114708097, -74.61680888518214, -79.35971237710655, -84.19381720546207, -89.0309568813179, -93.76626201506235, -98.30389147132843, -102.5674505604998, -106.5151070551369, -110.15736689630029, -113.54977209215946, -116.77255006938141, -119.91590432602138, -123.05412918661949, -126.21533904659755, -129.3788986714746, -132.48116030979827, -135.4201048130078, -138.0818803122765, -140.37954496631886, -142.27124486021165, -143.76482011578642, -144.91983255280093, -145.8269431169819, -146.58180184979122, -147.26501436671646, -147.91317707181136, -148.50822048069642, -148.98849189288472, -149.25934044222993, -149.21354979644676, -148.7532293966353, -147.8115072547339, -146.36170849743138, -144.40971973790528, -141.99642366484483, -139.18359548291608, -136.04124783130797, -132.64290795247504, -129.04910204029068, -125.30112513404919, -121.41858725546048, -117.39687761870707, -113.20699739739678, -108.8072644811206, -104.156447656929, -99.21782018147024, -93.97325026314, -88.44034651613146, -82.66910738693979, -76.73675159811216, -70.74815827746232, -64.80771664208692, -58.99526038848413, -53.36238076956079, -47.919624413813764, -42.6377795530664, -37.452466702622104, -32.26988720925385, -27.003665174490077, -21.601498763132117, -16.04863755737048, -10.383831203423101, -4.701113113597359, 0.8699954762405548, 6.175374153853591, 11.052903245357642, 15.36897795398104, 19.048384993321307, 22.06986650761941, 24.461968354310876, 26.306050404933533, 27.714137958707305, 28.806864902330297, 29.687800737856925, 30.421756456127678, 31.036197458573447, 31.513082024017137, 31.797648501696614, 31.83018608576985, 31.56136935477134, 30.96622141443909, 30.054865245421013, 28.870652498617673, 27.485958854891265, 25.98734308510105, 24.45560936638249, 22.949808399157426, 21.500608180252225, 20.117051961698316, 18.793661604240626, 17.515485506336926, 16.271205370286534, 15.060447931900732, 13.887907691249735, 12.761846078942794, 11.688537743129611, 10.664184315799067, 9.673777479833678, 8.69185998599029, 7.689722114362612, 6.644142712002756, 5.5489128542066375, 4.424808485325235, 3.3111142149681014, 2.2610891286393233, 1.335612785378006, 0.5877696454754735, 0.053521937854927204, -0.2567401384671376, -0.3557735512006922, -0.2784724612949696, -0.07853506282829614, 0.18256031818753327, 0.44304093460696903, 0.650039462448212, 0.764952579882793, 0.7689161694157858, 0.6737511596614851, 0.5172438995666861, 0.35911404243467393, 0.28301717392236014, 0.37633564061942204, 0.7076568226739712, 1.3075742720420016, 2.1621380128392493, 3.21400925917626, 4.3573630799991845, 5.455458641374711, 6.377350899742055, 7.023578026244541, 7.338794072654485, 7.322844297055978, 7.031320508649727, 6.558918697167101, 6.021565773032535, 5.5377714668214555, 5.20152775621661, 5.066449873655506, 5.145533050128437, 5.412328934970666, 5.811378465393334, 6.275243595277447, 6.731385290865964, 7.1106944337872395, 7.360007232480086, 7.447804576028288, 7.365010731281034, 7.124385711769431, 6.754884114074921, 6.298483828095357, 5.811034487227277, 5.350710368299195, 4.96862539394748, 4.703043389780561, 4.575043557818448, 4.587870364684006, 4.71955941472352, 4.9194045277860425, 5.118402915129714, 5.246131939783017, 5.24206719592353, 5.06924744570556, 4.726343259295357, 4.24718661239473, 3.6993376488674317, 3.175064946974269, 2.765805757169805, 2.5385817415799687, 2.5173537881648116, 2.6759449610368176, 2.9479262074497585, 3.237148717512281, 3.4341455551689926, 3.446421520800576, 3.227194291517243, 2.7817030989512874, 2.1614630528822882, 1.4523628951322545, 0.754094963516307, 0.1601843101240954, -0.264174228023232, -0.494983528989275, -0.5474694468927632, -0.4700905150379784, -0.3262189780626761, -0.17064050805013942, -0.04217573861347379, 0.03900903788751986, 0.073206117824693, 0.07126547583113041, 0.0434508455476319, 0.0010882962093266002, -0.043927100107675976, -0.08655377147080934, -0.12384424142226802, -0.1473349135451807, -0.14460265648910386, -0.105223179849256, -0.030575262284425975, 